vi "Main.vi"() -> ()   [LabVIEW 2015] (continued)
              n571 = case shown="False" w1144 {
                tunnel: w1143 -> [w1188 w1190]
                tunnel: [w1187 w1190] -> w1142
                frame False {
                  n572 = call "ShutterControl.vi"("error in"=w1188, "Shutter"=TRUE) -> ("error out"=w1187:errorcluster, "Status Indicator"=w1186:bool)  [unwired: 8 in]
                  n573 = local write "Shutter"(w1186) -> ()
                }
                frame True {
                }
              }
              n574 = call "ImageFrame.vi"("Tasks In"=w1184, "Vphases"=w1182, "Functions"=w1153, "error in"=w1142, "XYcoordinates"=w1183) -> ("Tasks Out"=w1180:T14, "Mixer AI Channels Data"=w1181:dbl[][], "DC AI Channel Date"=w1150:dbl[], "error out"=w1146:errorcluster)  [unwired: 6 in, 1 out]
              n575 = Unbundle By Name(w1146) -> ("status"=w1179:bool)
              n576 = Increment(x=w1157) -> (x+1=w1156:u32)
              n577 = call "Analysis.vi"("Functions"=w1153, "error in"=w1146, "Scan/Meas Parameters"=w1152, "Global Parameters"=w1151, "DC AI Channel Data"=w1150, "Mixer AI Channels Data"=w1181) -> ("AI Mix4 Data"=w1166:dbl[], "AI Mix3 Data"=w1163:dbl[], "AI Mix2 Data"=w1161:dbl[], "AI Mix1 Data"=w1159:dbl[], "AI DC Data"=w1177:dbl[], "error out"=w1145:errorcluster)
              n578 = Greater Or Equal?(x=w1156, y=w1171) -> (x >= y?=w1155:bool)
              n579 = Divide(x=w1156, y=w1171) -> (x/y=w1168:dbl)
              n580 = Compound Arithmetic op=OR(w1179, "Stop Measure", w1155) -> (w1178:bool)
              n581 = Reshape Array(w1159, w1158, w1158) -> (w1160:dbl[][])
              n582 = Reshape Array(w1161, w1158, w1158) -> (w1162:dbl[][])
              n583 = Reshape Array(w1163, w1158, w1158) -> (w1164:dbl[][])
              n584 = Reshape Array(w1166, w1158, w1158) -> (w1165:dbl[][])
              n585 = Reshape Array(w1177, w1158, w1158) -> (w1167:dbl[][])
              n586 = Multiply(x=w1168, y=100.0) -> (x*y=→"Meas Progress":dbl)
              n587 = local read "V_IF (0.5pi)"() -> (w1173:dbl[][])
              n588 = local read "V_IF (1.5pi)"() -> (w1175:dbl[][])
              n589 = local read "V_IF (pi)"() -> (w1174:dbl[][])
              n590 = local read "V_IF (0)"() -> (w1172:dbl[][])
              n591 = local read "V_DC"() -> (w1176:dbl[][])
              n592 = call "RunningAverage.vi"("New Image"=w1165, "# of Averages for the Old Image"=w1157, "Old Image"=w1175) -> ("Averaged Image"=w1138:dbl[][])  [unwired: 8 in]
              "V_IF (1.5pi)" <- w1138
              n593 = call "RunningAverage.vi"("New Image"=w1160, "# of Averages for the Old Image"=w1157, "Old Image"=w1172) -> ("Averaged Image"=w1141:dbl[][])  [unwired: 8 in]
              "V_IF (0)" <- w1141
              n594 = call "RunningAverage.vi"("New Image"=w1162, "# of Averages for the Old Image"=w1157, "Old Image"=w1173) -> ("Averaged Image"=w1140:dbl[][])  [unwired: 8 in]
              "V_IF (0.5pi)" <- w1140
              n595 = call "RunningAverage.vi"("New Image"=w1164, "# of Averages for the Old Image"=w1157, "Old Image"=w1174) -> ("Averaged Image"=w1139:dbl[][])  [unwired: 8 in]
              "V_IF (pi)" <- w1139
              n596 = call "RunningAverage.vi"("New Image"=w1167, "# of Averages for the Old Image"=w1157, "Old Image"=w1176) -> ("Averaged Image"=w1137:dbl[][])  [unwired: 8 in]
              "V_DC" <- w1137
              n597 = call "ShutterControl.vi"("error in"=w1145, "Shutter"=FALSE) -> ("error out"=w1147:errorcluster, "Status Indicator"=w1149:bool)  [unwired: 8 in]
              n598 = local write "Shutter"(w1149) -> ()
            }
            n599 = local read "[d13]"() -> (w1101:dbl)
            n600 = local read "[d24]"() -> (w1100:dbl)
            n601 = call "DAQClose.vi"("error in"=w1126, "Functions"=w1127, "Tasks In"=w1128, "DAQ Channels"=w1129) -> ("error out"=w1112:errorcluster)  [unwired: 7 in]
            n602 = local read "[M/B]"() -> (w1105:dbl)
            n603 = local read "[O_B]"() -> (w1104:dbl)
            n604 = call "GSCalculation.vi"("[d24]"=w1100, "[d13]"=w1101, "[O_B]"=w1104, "V_DC"=w1106, "[M/B]"=w1105, "V_IF (1.5pi)"=w1108, "V_IF (pi)"=w1109, "V_IF (0.5pi)"=w1110, "V_IF (0)"=w1111) -> ("S"=w1102:dbl[][], "G"=w1103:dbl[][])  [unwired: 1 in]
            "G Data" <- w1103
            "S Data" <- w1102
          }
          frame #2 {
            n605 = case shown="True" "Calculate Lifetimes and Phasors During Image Acquisition?" {
              tunnel: w1197 -> [w1200 w1229]
              tunnel: w1196 -> [_ w1221]
              tunnel: w1195 -> [_ w1208]
              tunnel: w1194 -> [_ w1207]
              tunnel: w1193 -> [_ w1206]
              tunnel: [w1200 w1201] -> w1192
              frame False {
                # "If need to be fast, e.g., 3D stack acquisition"
              }
              frame True {
                # "If do lifetime and other calcuations"
                n606 = Square(x=w1221) -> (x^2=w1239:i32)
                n607 = call "LifetimeCalculation.vi"("S"=w1206, "G"=w1207) -> ("DC&1w Lifetime"=w1230:dbl[][], "1w Lifetime"=w1231:dbl[][])  [unwired: 8 in]
                "1w Lifetime (s)" <- w1231
                "DC&1w Lifetime (s)" <- w1230
                n608 = control-ref of="1w Lifetime Hist"() -> (w1241:refnum<vi>)
                n609 = control-ref of="DC&1w Lifetime Hist"() -> (w1240:refnum<vi>)
                n610 = control-ref of="Lifetime Color Ramp"() -> (w1223:refnum<vi>)
                n611 = control-ref of="Phasor Plot"() -> (w1215:refnum<vi>)
                n612 = local read "Auto Scale?"() -> (w1203:bool)
                n613 = control-ref of="Composite Image"() -> (w1224:refnum<vi>)
                n614 = control-ref of="Image with Phasors"() -> (w1218:refnum<vi>)
                n615 = call "LifetimeHistogram.vi"("1w Lifetime"=w1231, "DC&1w Lifetime"=w1230, "1w reference"=w1241, "DC&1w reference"=w1240, "Max Lifetime (s)"="Max Lifetime (s)", "Min Lifetime (s)"="Min Lifetime (s)", "Data Size"=w1239, "error in (no error)"=w1229, "Bins"="Bins") -> ("error out"=w1225:errorcluster, "1w Lifetime Hist"=→"1w Lifetime Hist":T7, "DC&1w Lifetime Hist"=→"DC&1w Lifetime Hist":T7, "1w mean"=→"u_1w":dbl, "1w std"=→"std_1":dbl, "DC&1w mean"=→"u_01":dbl, "DC&1w std"=→"std_01":dbl)  [unwired: 4 in]
                n616 = case shown="\"1w Lifetime\", Default" "Lifetime Selection" {
                  tunnel: w1231 -> [w1245 _]
                  tunnel: w1230 -> [_ w1246]
                  tunnel: [w1245 w1246] -> w1228
                  frame "1w Lifetime", Default {
                  }
                  frame "DC&1w Lifetime" {
                  }
                }
                n617 = call "HSVCombIntensityLifetime.vi"("min_intensity"="Min Intensity", "Auto Scale?"=w1203, "max_intensity"="Max Intensity", "lifetime_max (s)"="Max Lifetime (s)", "lifetime_min (s)"="Min Lifetime (s)", "Lifetime image"=w1228, "Intensity image"=w1208) -> ("Min"=w1204:dbl, "Max"=w1205:dbl, "Lifetime Color Ramp"=→"Lifetime Color Ramp":i32[][], "HSV to RGB Picture"=→"Composite Image":picture)  [unwired: 1 in]
                n618 = call "Array2GrayPic.vi"("Pic Reference"=w1218, "Threshold (min)"=w1204, "Threshold (max)"=w1205, "Auto Scale?"=w1203, "Intensity"=w1208) -> ("Gray Picture"=→"Image with Phasors":picture)  [unwired: 6 in]
                n619 = local write "Max Intensity"(w1205) -> ()
                n620 = local write "Min Intensity"(w1204) -> ()
                n621 = property on="V_DC" class="IntGraph (strict)"(error in=w1225, "ZScale.Maximum"=w1205, "ZScale.Minimum"=w1204) -> (error out=w1222:errorcluster)  [unwired: 1 in, 1 out]
                n622 = call "CompositeProperties.vi"("Image Reference"=w1224, "Ramp Reference"=w1223, "Pixel Size"=w1221, "Max Lifetime (s)"="Max Lifetime (s)", "Min Lifetime (s)"="Min Lifetime (s)", "error in (no error)"=w1222) -> ("error out"=w1202:errorcluster)  [unwired: 13 in]
                n623 = call "DrawPhasorPlot.vi"("Intensity"=w1208, "G Data"=w1207, "S Data"=w1206, "Threshold (max)"=w1205, "Threshold (min)"=w1204, "error in"=w1202, "G_max"="G_max", "Auto Scale?"=w1203, "G_min"="G_min", "Phasor Grids"="Phasor Grids", "S_max"="S_max", "Reference"=w1215, "S_min"="S_min", "Phasor Colormap"="Phasor Colormap") -> ("Phasor Plot"=→"Phasor Plot":dbl[][], "error out"=w1201:errorcluster)  [unwired: 4 in]
              }
            }
          }
          frame #3 {
            w1254 = FALSE ("Fast Scan")
            n624 = Tick Count (ms)() -> (millisecond timer value=w1250:u32)
            n625 = local write "Measure"(w1254) -> ()
            n626 = local write "Stop Measure"(w1254) -> ()
            n627 = Subtract(x=w1250, y=w1249) -> (x-y=w1251:u32)
            n628 = To Double Precision Float(number=w1251) -> (double precision float=w1252:dbl)
            n629 = Divide(x=w1252, y=1000.0) -> (x/y=→"Actual Meas Time (s)":dbl)
          }
        }
      }
      event "Refresh": Value Change {
        n630 = event-data() -> ()  [unwired: 1 in, 1 out]
        n631 = flat-sequence {
          tunnel: [w1304] -> w1263
          tunnel: w1262 -> [w1304]
          tunnel: [w1302] -> w1260
          tunnel: w1259 -> [w1303]
          tunnel: w1263 -> [w1315]
          tunnel: [w1315] -> w1261
          tunnel: w1260 -> [w1314]
          tunnel: [w1314] -> w1258
          frame #0 {
            n632 = local read "Measurement Parameters"() -> (w1306:T4)
            n633 = Unbundle By Name(w1306) -> ("Pixel Size"=w1305:dbl)
            n634 = local read "G Data"() -> (w1308:dbl[][])
            n635 = local read "V_DC"() -> (w1310:dbl[][])
            n636 = local read "S Data"() -> (w1309:dbl[][])
            n637 = To Long Integer(number=w1305) -> (32bit integer=w1307:i32)
            n638 = Square(x=w1307) -> (x^2=w1301:i32)
            n639 = local read "Phasor Colormap"() -> (w1266:T8)
            n640 = local read "Max Lifetime (s)"() -> (w1295:dbl)
            n641 = local read "Min Lifetime (s)"() -> (w1294:dbl)
            n642 = control-ref of="Phasor Plot"() -> (w1265:refnum<vi>)
            n643 = control-ref of="Lifetime Color Ramp"() -> (w1275:refnum<vi>)
            n644 = call "LifetimeCalculation.vi"("S"=w1309, "G"=w1308) -> ("DC&1w Lifetime"=w1290:dbl[][], "1w Lifetime"=w1291:dbl[][])  [unwired: 8 in]
            n645 = local read "Bins"() -> (w1289:i32)
            n646 = control-ref of="1w Lifetime Hist"() -> (w1282:refnum<vi>)
            n647 = control-ref of="DC&1w Lifetime Hist"() -> (w1281:refnum<vi>)
            n648 = local read "Phasor Grids"() -> (w1267:i32)
            n649 = local read "Max Intensity"() -> (w1293:dbl)
            n650 = local read "Min Intensity"() -> (w1292:dbl)
            n651 = local read "Auto Scale?"() -> (w1297:bool)
            n652 = local read "G_max"() -> (w1271:dbl)
            n653 = local read "G_min"() -> (w1270:dbl)
            n654 = local read "S_max"() -> (w1269:dbl)
            n655 = local read "S_min"() -> (w1268:dbl)
            n656 = control-ref of="Image with Phasors"() -> (w1274:refnum<vi>)
            n657 = control-ref of="Composite Image"() -> (w1276:refnum<vi>)
            n658 = call "LifetimeHistogram.vi"("1w Lifetime"=w1291, "DC&1w Lifetime"=w1290, "1w reference"=w1282, "DC&1w reference"=w1281, "Max Lifetime (s)"=w1295, "Min Lifetime (s)"=w1294, "Data Size"=w1301, "error in (no error)"=w1303, "Bins"=w1289) -> ("error out"=w1299:errorcluster, "1w Lifetime Hist"=w1288:T7, "DC&1w Lifetime Hist"=w1287:T7, "1w mean"=w1286:dbl, "1w std"=w1285:dbl, "DC&1w mean"=w1284:dbl, "DC&1w std"=w1283:dbl)  [unwired: 4 in]
            n659 = local write "1w Lifetime (s)"(w1291) -> ()
            n660 = local write "DC&1w Lifetime (s)"(w1290) -> ()
            n661 = local write "1w Lifetime Hist"(w1288) -> ()
            n662 = local write "DC&1w Lifetime Hist"(w1287) -> ()
            n663 = local write "u_1w"(w1286) -> ()
            n664 = local write "std_1"(w1285) -> ()
            n665 = local write "u_01"(w1284) -> ()
            n666 = local write "std_01"(w1283) -> ()
            n667 = local read "Lifetime Selection"() -> (w1264:enum32{"1w Lifetime", "DC&1w Lifetime"})
            n668 = case shown="\"1w Lifetime\", Default" w1264 {
              tunnel: w1291 -> [w1311 _]
              tunnel: w1290 -> [_ w1312]
              tunnel: [w1311 w1312] -> w1300
              frame "1w Lifetime", Default {
              }
              frame "DC&1w Lifetime" {
              }
            }
            n669 = call "HSVCombIntensityLifetime.vi"("min_intensity"=w1292, "Auto Scale?"=w1297, "max_intensity"=w1293, "lifetime_max (s)"=w1295, "lifetime_min (s)"=w1294, "Lifetime image"=w1300, "Intensity image"=w1310) -> ("Min"=w1277:dbl, "Max"=w1278:dbl, "Lifetime Color Ramp"=w1279:i32[][], "HSV to RGB Picture"=w1280:picture)  [unwired: 1 in]
            n670 = call "Array2GrayPic.vi"("Pic Reference"=w1274, "Threshold (min)"=w1277, "Threshold (max)"=w1278, "Auto Scale?"=w1297, "Intensity"=w1310) -> ("Gray Picture"=w1273:picture)  [unwired: 6 in]
            n671 = local write "Image with Phasors"(w1273) -> ()
            n672 = property on="V_DC" class="IntGraph (strict)"(error in=w1299, "ZScale.Maximum"=w1278, "ZScale.Minimum"=w1277) -> (error out=w1298:errorcluster)  [unwired: 1 in, 1 out]
            n673 = call "CompositeProperties.vi"("Image Reference"=w1276, "Ramp Reference"=w1275, "Pixel Size"=w1307, "Max Lifetime (s)"=w1295, "Min Lifetime (s)"=w1294, "error in (no error)"=w1298) -> ("error out"=w1296:errorcluster)  [unwired: 13 in]
            n674 = call "DrawPhasorPlot.vi"("Intensity"=w1310, "G Data"=w1308, "S Data"=w1309, "Threshold (max)"=w1278, "Threshold (min)"=w1277, "error in"=w1296, "G_max"=w1271, "Auto Scale?"=w1297, "G_min"=w1270, "Phasor Grids"=w1267, "S_max"=w1269, "Reference"=w1265, "S_min"=w1268, "Phasor Colormap"=w1266) -> ("Phasor Plot"=w1272:dbl[][], "error out"=w1302:errorcluster)  [unwired: 4 in]
            n675 = local write "Phasor Plot"(w1272) -> ()
            n676 = local write "Composite Image"(w1280) -> ()
            n677 = local write "Lifetime Color Ramp"(w1279) -> ()
            n678 = local write "Max Intensity"(w1278) -> ()
            n679 = local write "Min Intensity"(w1277) -> ()
          }
          frame #1 {
            n680 = local write "Refresh"(FALSE ("Fast Scan")) -> ()
          }
        }
      }
      event "Z-Stack Measure": Value Change {
        n681 = event-data() -> ()  [unwired: 1 in, 1 out]
        n682 = local read "Current Slice"() -> (w1324:i32)
        n683 = Divide(x=w1324, y="Z Slice Number") -> (x/y=w1332:dbl)
        n684 = Greater Or Equal?(x=w1324, y="Z Slice Number") -> (x >= y?=w1325:bool)
        n685 = Multiply(x=w1332, y=100.0) -> (x*y=→"Stack Progress":dbl)
        n686 = Equal To 0?(x=w1324) -> (x = 0?=w1323:bool)
        n687 = case shown="False" w1323 {
          tunnel: w1334 -> [w1380 w1407]
          tunnel: w1335 -> [w1379 w1408]
          tunnel: [w1378 w1406] -> w1328
          tunnel: [w1377 w1405] -> w1326
          tunnel: w1325 -> [w1373 _]
          tunnel: [FALSE ("Stop Stack Measure") w1400] -> w1316
          frame False {
            # "Continue measurement , move stage"
            n688 = local read "3D Intensity"() -> (w1374:dbl[][][])
            n689 = local read "G Data"() -> (w1372:dbl[][])
            n690 = local read "S Data"() -> (w1371:dbl[][])
            n691 = local read "V_DC"() -> (w1376:dbl[][])
            n692 = local read "3D G"() -> (w1368:dbl[][][])
            n693 = local read "3D S"() -> (w1367:dbl[][][])
            n694 = case shown="False" w1373 {
              tunnel: w1380 -> [w1396 w1397]
              tunnel: w1379 -> [w1395 w1398]
              tunnel: [w1383 w1398] -> w1378
              tunnel: [w1381 w1397] -> w1377
              frame False {
                # "Moves up by 1 step defined by \nthe 'C' command"
                n695 = Number To Decimal String(number="Z Slice Size (.1um)") -> (decimal integer string=w1389:string)  [unwired: 1 in]
                n696 = Concatenate Strings("C" ("string"), "," ("string"), w1389, "\r", "U" ("string")) -> (w1386:string)
                n697 = VISA Write(VISA resource name=w1395, write buffer=w1386, error in (no error)=w1396) -> (VISA resource name out=w1393:refnum<visa-resource-name>, error out=w1392:errorcluster)  [unwired: 1 out]
                n698 = VISA Read(VISA resource name=w1393, byte count=u32 256, error in (no error)=w1392) -> (VISA resource name out=w1384:refnum<visa-resource-name>, error out=w1382:errorcluster)  [unwired: 2 out]
                n699 = VISA Clear(VISA resource name=w1384, error in (no error)=w1382) -> (VISA resource name out=w1383:refnum<visa-resource-name>, error out=w1381:errorcluster)
              }
              frame True {
              }
            }
            n700 = Build Array (concatenate)(w1374, w1376) -> (→"3D Intensity":dbl[][][])
            n701 = Build Array (concatenate)(w1368, w1372) -> (→"3D G":dbl[][][])
            n702 = Build Array (concatenate)(w1367, w1371) -> (→"3D S":dbl[][][])
          }
          frame True {
            # "Beginning the measurment, record current Z position"
            n703 = local read "3D Time-Lapse Measure"() -> (w1399:bool)
            n704 = case shown="False" w1399 {
              tunnel: [w1413 TRUE ("T button?")] -> w1401
              frame False {
                n705 = Two Button Dialog(message="Discard Previous Stack?") -> (T button?=w1413:bool)  [unwired: 2 in]
              }
              frame True {
              }
            }
            n706 = local write "Calculate Lifetimes and Phasors During Image Acquisition?"(FALSE ("Calculate Lifetimes and Phasors During Image Acquisition?")) -> ()
            n707 = VISA Write(VISA resource name=w1408, write buffer="PZ" ("string"), error in (no error)=w1407) -> (VISA resource name out=w1410:refnum<visa-resource-name>, error out=w1411:errorcluster)  [unwired: 1 out]
            n708 = VISA Read(VISA resource name=w1410, byte count=u32 256, error in (no error)=w1411) -> (VISA resource name out=w1406:refnum<visa-resource-name>, read buffer=w1404:string, error out=w1405:errorcluster)  [unwired: 1 out]
            n709 = case shown="True" w1401 {
              tunnel: [TRUE ("Stop Stack Measure") FALSE ("Stop Stack Measure")] -> w1400
              frame False {
              }
              frame True {
                w1418 = dbl[][][] [] ("3D Intensity (BT)")
                n710 = local write "3D Intensity"(w1418) -> ()
                n711 = local write "3D G"(w1418) -> ()
                n712 = local write "3D S"(w1418) -> ()
              }
            }
            n713 = Decimal String To Number(string=w1404) -> (number=→"Initial Z Pos (.1um)":i32)  [unwired: 2 in, 1 out]
          }
        }
        n714 = Compound Arithmetic op=OR(w1325, "Stop Stack Measure", w1316) -> (w1329:bool)
        n715 = case shown="True" w1329 {
          tunnel: w1328 -> [w1342 w1346]
          tunnel: w1326 -> [w1337 w1345]
          tunnel: [w1342 w1351] -> w1322
          tunnel: [w1339 w1347] -> w1320
          tunnel: w1324 -> [w1341 _]
          frame False {
            n716 = Increment(x=w1341) -> (x+1=→"Current Slice":i32)
            n717 = property on="Measure" class="Bool (strict)"(error in=w1337, "Val(Sgnl)"=TRUE ("Value (Signaling)")) -> (error out=w1336:errorcluster)  [unwired: 1 in, 1 out]
            n718 = property on="Z-Stack Measure" class="Bool (strict)"(error in=w1336, "Val(Sgnl)"=TRUE ("Value (Signaling)")) -> (error out=w1339:errorcluster)  [unwired: 1 in, 1 out]
          }
          frame True {
            w1350 = FALSE ("Fast Scan")
            n719 = local read "Initial Z Pos (.1um)"() -> (w1360:i32)
            n720 = local read "3D Time-Lapse Measure"() -> (w1349:bool)
            n721 = local write "Calculate Lifetimes and Phasors During Image Acquisition?"(TRUE ("Calculate Lifetimes and Phasors During Image Acquisition?")) -> ()
            n722 = local write "Stop Stack Measure"(w1350) -> ()
            n723 = local write "Z-Stack Measure"(w1350) -> ()
            n724 = local write "Current Slice"(0 ("Current Slice")) -> ()
            n725 = Number To Decimal String(number=w1360) -> (decimal integer string=w1357:string)  [unwired: 1 in]
            n726 = Concatenate Strings("GZ" ("string"), "," ("string"), w1357) -> (w1359:string)
            n727 = VISA Write(VISA resource name=w1346, write buffer=w1359, error in (no error)=w1345) -> (VISA resource name out=w1354:refnum<visa-resource-name>, error out=w1355:errorcluster)  [unwired: 1 out]
            n728 = VISA Read(VISA resource name=w1354, byte count=u32 256, error in (no error)=w1355) -> (VISA resource name out=w1351:refnum<visa-resource-name>, error out=w1348:errorcluster)  [unwired: 2 out]
            n729 = case shown="True" w1349 {
              tunnel: w1348 -> [w1361 w1363]
              tunnel: [w1361 w1362] -> w1347
              frame False {
              }
              frame True {
                w1364 = TRUE ("Value (Signaling)")
                n730 = property on="Save 3D Stacks" class="Bool (strict)"(error in=w1363, "Val(Sgnl)"=w1364) -> (error out=w1365:errorcluster)  [unwired: 1 in, 1 out]
                n731 = property on="3D Time-Lapse Measure" class="Bool (strict)"(error in=w1365, "Val(Sgnl)"=w1364) -> (error out=w1362:errorcluster)  [unwired: 1 in, 1 out]
              }
            }
          }
        }
        n732 = VISA Clear(VISA resource name=w1322, error in (no error)=w1320) -> (VISA resource name out=w1321:refnum<visa-resource-name>, error out=w1319:errorcluster)
      }
      event "3D Stack to Show", "Slice Slider": Value Change {
        n733 = event-data() -> ()  [unwired: 1 in, 1 out]
        n734 = local read "3D Intensity"() -> (w1441:dbl[][][])
        n735 = local read "Max Lifetime (s)"() -> (w1443:dbl)
        n736 = local read "Min Lifetime (s)"() -> (w1442:dbl)
        n737 = case shown="False" "Auto Scale?" {
          tunnel: w1441 -> [_ w1461]
          tunnel: [w1458 w1460] -> w1440
          tunnel: [w1457 w1459] -> w1439
          frame False {
            n738 = local read "Max Intensity"() -> (w1458:dbl)
            n739 = local read "Min Intensity"() -> (w1457:dbl)
          }
          frame True {
            n740 = Array Max & Min(array=w1461) -> (max value=w1460:dbl, min value=w1459:dbl)  [unwired: 2 out]
          }
        }
        n741 = local read "3D G"() -> (w1425:dbl[][][])
        n742 = local read "3D S"() -> (w1424:dbl[][][])
        n743 = control-ref of="Slice of 3D Stack"() -> (w1426:refnum<vi>)
        n744 = Multiply(x=80000000.0, y=6.283185307179586) -> (x*y=w1421:dbl)
        n745 = case shown="\"Intensity 3D\", Default" "3D Stack to Show" {
          tunnel: "Slice Slider" -> [w1471 w1484 w1500 w1517 w1538 w1558 w1577]
          tunnel: [w1469 w1483 w1499 w1518 w1537 w1561 w1580] -> w1444
          tunnel: w1443 -> [_ w1479 w1496 w1510 w1528 _ _]
          tunnel: w1442 -> [_ w1478 w1495 w1509 w1521 _ _]
          tunnel: w1441 -> [w1468 _ _ w1516 w1536 w1562 w1581]
          tunnel: w1440 -> [w1464 _ _ w1513 w1531 w1547 w1572]
          tunnel: w1439 -> [w1463 _ _ w1512 w1530 w1546 w1571]
          tunnel: [w1462 w1477 w1494 w1507 w1533 w1542 w1574] -> w1428
          tunnel: w1426 -> [w1466 w1481 w1493 w1515 w1534 w1543 w1576]
          tunnel: w1425 -> [_ w1475 w1490 w1505 w1523 w1560 w1579]
          tunnel: w1424 -> [_ w1474 _ w1504 _ w1559 w1578]
          tunnel: w1421 -> [_ w1473 w1487 w1503 w1522 _ _]
          frame "Intensity 3D", Default {
            n746 = Array Size(array=w1468) -> (size(s)=w1470:i32[])
            n747 = Index Array(array=w1468, index (dim 0)=w1471) -> (element=w1467:dbl[][])  [unwired: 2 in]
            n748 = Index Array(array=w1470) -> (element=w1469:i32)  [unwired: 1 in]
            n749 = call "Array2GrayPic.vi"("Pic Reference"=w1466, "Threshold (min)"=w1463, "Threshold (max)"=w1464, "Auto Scale?"=FALSE, "Intensity"=w1467) -> ("Gray Picture"=w1462:picture)  [unwired: 6 in]
          }
          frame "1w Lifetime 3D" {
            n750 = Divide(x=w1474, y=w1475) -> (x/y=w1476:dbl[][][])
            n751 = Divide(x=w1476, y=w1473) -> (x/y=w1472:dbl[][][])
            n752 = Array Size(array=w1472) -> (size(s)=w1485:i32[])
            n753 = Index Array(array=w1472, index (dim 0)=w1484) -> (element=w1480:dbl[][])  [unwired: 2 in]
            n754 = Index Array(array=w1485) -> (element=w1483:i32)  [unwired: 1 in]
            n755 = call "Array2GrayPic.vi"("Pic Reference"=w1481, "Threshold (min)"=w1478, "Threshold (max)"=w1479, "Auto Scale?"=FALSE, "Intensity"=w1480) -> ("Gray Picture"=w1477:picture)  [unwired: 6 in]
          }
          frame "DC&1w Lifetime 3D" {
            n756 = Divide(x=1.0, y=w1490) -> (x/y=w1489:dbl[][][])
            n757 = Decrement(x=w1489) -> (x-1=w1492:dbl[][][])
            n758 = Square Root(x=w1492) -> (sqrt(x)=w1488:dbl[][][])
            n759 = Divide(x=w1488, y=w1487) -> (x/y=w1486:dbl[][][])
            n760 = Array Size(array=w1486) -> (size(s)=w1501:i32[])
            n761 = Index Array(array=w1486, index (dim 0)=w1500) -> (element=w1497:dbl[][])  [unwired: 2 in]
            n762 = Index Array(array=w1501) -> (element=w1499:i32)  [unwired: 1 in]
            n763 = call "Array2GrayPic.vi"("Pic Reference"=w1493, "Threshold (min)"=w1495, "Threshold (max)"=w1496, "Auto Scale?"=FALSE, "Intensity"=w1497) -> ("Gray Picture"=w1494:picture)  [unwired: 6 in]
          }
          frame "1w Composite 3D" {
            n764 = Divide(x=w1504, y=w1505) -> (x/y=w1506:dbl[][][])
            n765 = Divide(x=w1506, y=w1503) -> (x/y=w1502:dbl[][][])
            n766 = Index Array(array=w1502, index (dim 0)=w1517) -> (element=w1511:dbl[][])  [unwired: 2 in]
            n767 = Index Array(array=w1516, index (dim 0)=w1517) -> (element=w1514:dbl[][])  [unwired: 2 in]
            n768 = Array Size(array=w1516) -> (size(s)=w1519:i32[])
            n769 = Index Array(array=w1519) -> (element=w1518:i32)  [unwired: 1 in]
            n770 = call "Array2HSVColorPic.vi"("Intensity"=w1514, "Threshold (max)"=w1513, "Threshold (min)"=w1512, "Lifetime"=w1511, "lifetime_max (s)"=w1510, "lifetime_min (s)"=w1509, "Pic Reference"=w1515, "Auto Scale?"=FALSE) -> ("Gray Picture"=w1507:picture)  [unwired: 11 in]
          }
          frame "DC&1w Composite 3D" {
            n771 = Divide(x=1.0, y=w1523) -> (x/y=w1525:dbl[][][])
            n772 = Decrement(x=w1525) -> (x-1=w1527:dbl[][][])
            n773 = Square Root(x=w1527) -> (sqrt(x)=w1524:dbl[][][])
            n774 = Divide(x=w1524, y=w1522) -> (x/y=w1520:dbl[][][])
            n775 = Index Array(array=w1520, index (dim 0)=w1538) -> (element=w1529:dbl[][])  [unwired: 2 in]
            n776 = Index Array(array=w1536, index (dim 0)=w1538) -> (element=w1532:dbl[][])  [unwired: 2 in]
            n777 = Array Size(array=w1536) -> (size(s)=w1539:i32[])
            n778 = Index Array(array=w1539) -> (element=w1537:i32)  [unwired: 1 in]
            n779 = call "Array2HSVColorPic.vi"("Intensity"=w1532, "Threshold (max)"=w1531, "Threshold (min)"=w1530, "Lifetime"=w1529, "lifetime_max (s)"=w1528, "lifetime_min (s)"=w1521, "Pic Reference"=w1534, "Auto Scale?"=FALSE) -> ("Gray Picture"=w1533:picture)  [unwired: 11 in]
          }
          frame "Phasor 3D" {
            # "Transpose"
            n780 = Array Size(array=w1562) -> (size(s)=w1563:i32[])
            n781 = Index Array(array=w1559, index (dim 0)=w1558) -> (element=w1548:dbl[][])  [unwired: 2 in]
            n782 = Index Array(array=w1560, index (dim 0)=w1558) -> (element=w1549:dbl[][])  [unwired: 2 in]
            n783 = Index Array(array=w1562, index (dim 0)=w1558) -> (element=w1550:dbl[][])  [unwired: 2 in]
            n784 = Index Array(array=w1563) -> (element=w1561:i32)  [unwired: 1 in]
            n785 = local read "Phasor Colormap"() -> (w1551:T8)
            n786 = local read "G_max"() -> (w1557:dbl)
            n787 = local read "G_min"() -> (w1556:dbl)
            n788 = local read "S_max"() -> (w1555:dbl)
            n789 = local read "S_min"() -> (w1554:dbl)
            n790 = control-ref of="Phasor Plot"() -> (w1552:refnum<vi>)
            n791 = local read "Phasor Grids"() -> (w1553:i32)
            n792 = call "DrawPhasorPlot.vi"("Intensity"=w1550, "G Data"=w1549, "S Data"=w1548, "Threshold (max)"=w1547, "Threshold (min)"=w1546, "G_max"=w1557, "Auto Scale?"=FALSE, "G_min"=w1556, "Phasor Grids"=w1553, "S_max"=w1555, "Reference"=w1552, "S_min"=w1554, "Phasor Colormap"=w1551) -> ("Phasor Plot"=w1540:dbl[][])  [unwired: 5 in, 1 out]
            n793 = Transpose 2D Array(2D array=w1540) -> (transposed array=w1541:dbl[][])
            n794 = call "Array2GrayPic.vi"("Pic Reference"=w1543, "Auto Scale?"=TRUE, "Intensity"=w1541) -> ("Gray Picture"=w1542:picture)  [unwired: 8 in]
          }
          frame "Overlap 3D" {
            n795 = Array Size(array=w1581) -> (size(s)=w1582:i32[])
            n796 = Index Array(array=w1581, index (dim 0)=w1577) -> (element=w1575:dbl[][])  [unwired: 2 in]
            n797 = Index Array(array=w1578, index (dim 0)=w1577) -> (element=w1569:dbl[][])  [unwired: 2 in]
            n798 = Index Array(array=w1579, index (dim 0)=w1577) -> (element=w1570:dbl[][])  [unwired: 2 in]
            n799 = Index Array(array=w1582) -> (element=w1580:i32)  [unwired: 1 in]
            n800 = local read "ROI Cluster"() -> (w1568:T9)
            n801 = Unbundle(w1568) -> (w1567:bool[], w1566:dbl[], w1565:cluster{dbl, dbl}[], w1564:u32[])
            n802 = call "PhasorROI2IMG.vi"("Intensity"=w1575, "Auto Scale?"=FALSE, "Threshold (max)"=w1572, "Threshold (min)"=w1571, "G Data"=w1570, "S Data"=w1569, "Pic Reference"=w1576, "ROI? array"=w1567, "Radius array"=w1566, "Center array"=w1565, "Color array"=w1564) -> ("new picture"=w1574:picture)  [unwired: 8 in]
          }
        }
        "Slice of 3D Stack" <- w1428
        "Number of Slices" <- w1444
        n803 = local read "Measurement Parameters"() -> (w1438:T4)
        n804 = property on="Slice of 3D Stack" class="Pict"(error in=w1432) -> (error out=w1431:errorcluster, "Draw Area Size"=w1436:T16)  [unwired: 1 in, 1 out]
        n805 = Unbundle By Name(w1436) -> ("Width"=w1433:u32)
        n806 = Unbundle By Name(w1438) -> ("Pixel Size"=w1429:dbl)
        n807 = To Single Precision Float(number=w1433) -> (single precision float=w1435:sgl)
        n808 = To Single Precision Float(number=w1429) -> (single precision float=w1434:sgl)
        n809 = Divide(x=w1435, y=w1434) -> (x/y=w1437:sgl)
        n810 = property on="Slice of 3D Stack" class="Pict"(error in=w1431, "ZoomFactor"=w1437) -> (error out=w1430:errorcluster)  [unwired: 1 in, 1 out]
        n811 = Increment(x="Slice Slider") -> (x+1=w1450:i32)
        n812 = Number To Decimal String(number=w1450) -> (decimal integer string=w1448:string)  [unwired: 1 in]
        n813 = Number To Decimal String(number=w1444) -> (decimal integer string=w1453:string)  [unwired: 1 in]
        n814 = property on="Slice Slider" class="Scroll (strict)"(error in=w1430, "DocMax"=w1444) -> (error out=w1447:errorcluster)  [unwired: 1 in, 1 out]
        n815 = Concatenate Strings("Slice #: " ("string"), w1448, "/" ("string"), w1453) -> (→"Slice Display":string)
        n816 = property on="Slice Slider" class="Scroll (strict)"(error in=w1447, "DocMin"=0.0 ("Doc Min")) -> (error out=w1446:errorcluster)  [unwired: 1 in, 1 out]
      }
      event "Save 3D Stacks": Value Change {
        # "Always save raw data for 3D"
        n817 = event-data() -> ()  [unwired: 1 in, 1 out]
        n818 = local read "3D Intensity"() -> (w1611:dbl[][][])
        n819 = local read "Current 3D Time-Lapse Meas"() -> (w1613:i32)
        n820 = local read "Crop Pixels"() -> (w1598:u16)
        n821 = local read "3D G"() -> (w1603:dbl[][][])
        n822 = local read "3D S"() -> (w1601:dbl[][][])
        n823 = case shown="True" TRUE {
          tunnel: [w1617 w1619] -> w1610
          tunnel: [w1616 w1618] -> w1609
          tunnel: w1611 -> [_ w1620]
          frame False {
            n824 = local read "Max Intensity"() -> (w1617:dbl)
            n825 = local read "Min Intensity"() -> (w1616:dbl)
          }
          frame True {
            n826 = Array Max & Min(array=w1620) -> (max value=w1619:dbl, min value=w1618:dbl)  [unwired: 2 out]
          }
        }
        n827 = case shown="True" "Current Directory (3D)?" {
          tunnel: ["Save Directory (3D)" w1622] -> w1599
          frame False {
          }
          frame True {
            n828 = Current VI's Path() -> (path=w1623:path)
            n829 = Strip Path(path=w1623) -> (stripped path=w1622:path)  [unwired: 1 out]
          }
        }
        n830 = Number To Decimal String(number=w1613) -> (decimal integer string=w1596:string)  [unwired: 1 in]
        n831 = call "Save3DStack.vi"("Experiment Name"="Experiment Name (3D)", "Identify Name"="I" ("string"), "3D Data"=w1611, "matrix_max"=w1610, "matrix_min"=w1609, "error in"=w1608, "File Name"="File Name (3D)", "Index Name"=w1596, "path"=w1599, "Specify Range?"=TRUE ("Bound Pixel Value?"), "Enable?"=TRUE, "Crop Pixels"=w1598, "Time Stamp?"=FALSE ("Enable?")) -> ("error out"=w1604:errorcluster)  [unwired: 5 in, 1 out]
        n832 = call "Save3DStack.vi"("Experiment Name"="Experiment Name (3D)", "Identify Name"="G" ("string"), "3D Data"=w1603, "error in"=w1604, "File Name"="File Name (3D)", "Index Name"=w1596, "path"=w1599, "Specify Range?"=FALSE ("Bound Pixel Value?"), "Enable?"=TRUE, "Crop Pixels"=w1598, "Time Stamp?"=FALSE ("Enable?")) -> ("error out"=w1591:errorcluster)  [unwired: 7 in, 1 out]
        n833 = call "Save3DStack.vi"("Experiment Name"="Experiment Name (3D)", "Identify Name"="S" ("string"), "3D Data"=w1601, "error in"=w1591, "File Name"="File Name (3D)", "Index Name"=w1596, "path"=w1599, "Specify Range?"=FALSE ("Bound Pixel Value?"), "Enable?"=TRUE, "Crop Pixels"=w1598, "Time Stamp?"=FALSE ("Enable?")) -> ("error out"=w1602:errorcluster)  [unwired: 7 in, 1 out]
        n834 = flat-sequence {
          tunnel: w1602 -> [w1625]
          tunnel: [w1625] -> w1586
          frame #0 {
            n835 = local write "Save 3D Stacks"(FALSE ("Save 3D Stacks")) -> ()
          }
        }
      }
      event "2D Time-Lapse Measure": Value Change {
        n836 = event-data() -> ()  [unwired: 1 in, 1 out]
        n837 = local read "Current 2D Time-Lapse Meas"() -> (w1631:i32)
        n838 = Divide(x=w1631, y="Total 2D Time-Lapse Meas") -> (x/y=w1636:dbl)
        n839 = Greater Or Equal?(x=w1631, y="Total 2D Time-Lapse Meas") -> (x >= y?=w1637:bool)
        n840 = Multiply(x=w1636, y=100.0) -> (x*y=→"2D Time-Lapse Progress":dbl)
        n841 = Compound Arithmetic op=OR(w1637, "Stop 2D Time-Lapse") -> (w1633:bool)
        n842 = case shown="False" w1633 {
          tunnel: w1631 -> [w1642 _]
          tunnel: w1629 -> [w1643 w1662]
          tunnel: [w1644 w1662] -> w1628
          frame False {
            w1645 = TRUE ("Value (Signaling)")
            n843 = Equal To 0?(x=w1642) -> (x = 0?=w1641:bool)
            n844 = case shown="False" w1641 {
              tunnel: [w1652 w1661] -> w1640
              tunnel: w1643 -> [w1652 w1661]
              frame False {
                n845 = while {
                  stop <- w1654 stop-if-true
                  n846 = local read "Time Stamp (s)"() -> (w1658:dbl)
                  n847 = Get Date/Time In Seconds() -> (seconds since 1Jan1904=w1660:timestamp)
                  n848 = local read "Stop 2D Time-Lapse"() -> (w1653:bool)
                  n849 = To Double Precision Float(number=w1660) -> (double precision float=w1659:dbl)
                  n850 = Subtract(x=w1659, y=w1658) -> (x-y=w1657:dbl)
                  "Time Elapse (s)" <- w1657
                  n851 = Greater Or Equal?(x=w1657, y="2D Time-Lapse Interval (s)") -> (x >= y?=w1655:bool)
                  n852 = Compound Arithmetic op=OR(w1655, w1653) -> (w1654:bool)
                }
              }
              frame True {
              }
            }
            n853 = Increment(x=w1642) -> (x+1=→"Current 2D Time-Lapse Meas":i32)
            n854 = flat-sequence {
              tunnel: [w1651] -> w1639
              tunnel: w1640 -> [w1651]
              frame #0 {
                n855 = Get Date/Time In Seconds() -> (seconds since 1Jan1904=w1649:timestamp)
                n856 = To Double Precision Float(number=w1649) -> (double precision float=→"Time Stamp (s)":dbl)
              }
            }
            n857 = property on="Measure" class="Bool (strict)"(error in=w1639, "Val(Sgnl)"=w1645) -> (error out=w1647:errorcluster)  [unwired: 1 in, 1 out]
            n858 = property on="Save 2D Images" class="Bool (strict)"(error in=w1647, "Val(Sgnl)"=w1645) -> (error out=w1646:errorcluster)  [unwired: 1 in, 1 out]
            n859 = property on="2D Time-Lapse Measure" class="Bool (strict)"(error in=w1646, "Val(Sgnl)"=w1645) -> (error out=w1644:errorcluster)  [unwired: 1 in, 1 out]
          }
          frame True {
            w1663 = FALSE ("2D Time-Lapse Measure")
            n860 = local write "Current 2D Time-Lapse Meas"(0 ("Current Slice")) -> ()
            n861 = local write "2D Time-Lapse Measure"(w1663) -> ()
            n862 = local write "Stop 2D Time-Lapse"(w1663) -> ()
          }
        }
      }
      event "3D Time-Lapse Measure": Value Change {
        n863 = event-data() -> ()  [unwired: 1 in, 1 out]
        n864 = local read "Current 3D Time-Lapse Meas"() -> (w1675:i32)
        n865 = Divide(x=w1675, y="Total 3D Time-Lapse Meas") -> (x/y=w1669:dbl)
        n866 = Greater Or Equal?(x=w1675, y="Total 3D Time-Lapse Meas") -> (x >= y?=w1673:bool)
        n867 = Multiply(x=w1669, y=100.0) -> (x*y=→"3D Time-Lapse Progress":dbl)
        n868 = Compound Arithmetic op=OR(w1673, "Stop 3D Time-Lapse") -> (w1676:bool)
        n869 = case shown="False" w1676 {
          tunnel: w1675 -> [w1684 _]
          tunnel: w1668 -> [w1681 w1699]
          tunnel: [w1678 w1699] -> w1667
          frame False {
            n870 = Equal To 0?(x=w1684) -> (x = 0?=w1683:bool)
            n871 = case shown="False" w1683 {
              tunnel: w1681 -> [w1689 w1698]
              tunnel: [w1689 w1698] -> w1680
              frame False {
                n872 = while {
                  stop <- w1690 stop-if-true
                  n873 = local read "Time Stamp (s)"() -> (w1695:dbl)
                  n874 = Get Date/Time In Seconds() -> (seconds since 1Jan1904=w1697:timestamp)
                  n875 = local read "Stop 3D Time-Lapse"() -> (w1691:bool)
                  n876 = To Double Precision Float(number=w1697) -> (double precision float=w1696:dbl)
                  n877 = Subtract(x=w1696, y=w1695) -> (x-y=w1693:dbl)
                  n878 = Greater Or Equal?(x=w1693, y="3D Time-Lapse Interval (s)") -> (x >= y?=w1694:bool)
                  n879 = local write "Time Elapse (s)"(w1693) -> ()
                  n880 = Compound Arithmetic op=OR(w1694, w1691) -> (w1690:bool)
                }
              }
              frame True {
              }
            }
            n881 = Increment(x=w1684) -> (x+1=→"Current 3D Time-Lapse Meas":i32)
            n882 = flat-sequence {
              tunnel: [w1686] -> w1679
              tunnel: w1680 -> [w1686]
              frame #0 {
                n883 = Get Date/Time In Seconds() -> (seconds since 1Jan1904=w1688:timestamp)
                n884 = To Double Precision Float(number=w1688) -> (double precision float=w1687:dbl)
                n885 = local write "Time Stamp (s)"(w1687) -> ()
              }
            }
            n886 = property on="Z-Stack Measure" class="Bool (strict)"(error in=w1679, "Val(Sgnl)"=TRUE ("Value (Signaling)")) -> (error out=w1678:errorcluster)  [unwired: 1 in, 1 out]
          }
          frame True {
            w1700 = FALSE ("2D Time-Lapse Measure")
            n887 = local write "Current 3D Time-Lapse Meas"(0 ("Current Slice")) -> ()
            n888 = local write "3D Time-Lapse Measure"(w1700) -> ()
            n889 = local write "Stop 3D Time-Lapse"(w1700) -> ()
          }
        }
      }
      event "Lifetime Selection", "Min Lifetime (s)", "Max Lifetime (s)", "Bins", "Max Intensity", "Min Intensity", "Auto Scale?": Value Change {
        w1717 = 100.0 ("y")
        n890 = event-data() -> ()  [unwired: 1 in, 1 out]
        n891 = local read "Lifetime Selection"() -> (w1743:enum32{"1w Lifetime", "DC&1w Lifetime"})
        n892 = case shown="\"DC&1w Lifetime\"" w1743 {
          tunnel: [w1745 w1746] -> w1738
          frame "1w Lifetime", Default {
            n893 = local read "1w Lifetime (s)"() -> (w1745:dbl[][])
          }
          frame "DC&1w Lifetime" {
            n894 = local read "DC&1w Lifetime (s)"() -> (w1746:dbl[][])
          }
        }
        n895 = local read "Auto Scale?"() -> (w1735:bool)
        n896 = local read "Max Lifetime (s)"() -> (w1712:dbl)
        n897 = local read "Max Intensity"() -> (w1737:dbl)
        n898 = local read "Min Lifetime (s)"() -> (w1711:dbl)
        n899 = local read "Min Intensity"() -> (w1736:dbl)
        n900 = local read "V_DC"() -> (w1727:dbl[][])
        n901 = call "HSVCombIntensityLifetime.vi"("min_intensity"=w1736, "Auto Scale?"=w1735, "max_intensity"=w1737, "lifetime_max (s)"=w1712, "lifetime_min (s)"=w1711, "Lifetime image"=w1738, "Intensity image"=w1727) -> ("Min"=w1704:dbl, "Max"=w1705:dbl, "Lifetime Color Ramp"=w1742:i32[][], "HSV to RGB Picture"=w1741:picture)  [unwired: 1 in]
        n902 = Array Max & Min(array=w1727) -> (max value=w1726:dbl, min value=w1724:dbl)  [unwired: 2 out]
        n903 = local write "Lifetime Color Ramp"(w1742) -> ()
        n904 = local write "Composite Image"(w1741) -> ()
        n905 = Subtract(x=w1704, y=w1724) -> (x-y=w1723:dbl)
        n906 = Subtract(x=w1726, y=w1724) -> (x-y=w1722:dbl)
        n907 = Subtract(x=w1705, y=w1724) -> (x-y=w1725:dbl)
        n908 = control-ref of="V_DC"() -> (w1706:refnum<vi>)
        n909 = Divide(x=w1725, y=w1722) -> (x/y=w1721:dbl)
        n910 = Divide(x=w1723, y=w1722) -> (x/y=w1719:dbl)
        n911 = Multiply(x=w1721, y=w1717) -> (x*y=w1720:dbl)
        n912 = Multiply(x=w1719, y=w1717) -> (x*y=w1718:dbl)
        n913 = local write "Max Intensity"(w1705) -> ()
        n914 = local write "Min Intensity"(w1704) -> ()
        n915 = property class="IntGraph (strict)"(reference=w1706, error in=w1708, "ZScale.Maximum"=w1705, "ZScale.Minimum"=w1704) -> (error out=w1707:errorcluster)  [unwired: 1 out]
        n916 = local write "Max (%)"(w1720) -> ()
        n917 = local write "Min (%)"(w1718) -> ()
        n918 = local read "Measurement Parameters"() -> (w1740:T4)
        n919 = local read "Bins"() -> (w1730:i32)
        n920 = local read "1w Lifetime (s)"() -> (w1734:dbl[][])
        n921 = local read "DC&1w Lifetime (s)"() -> (w1733:dbl[][])
        n922 = Unbundle By Name(w1740) -> ("Pixel Size"=w1739:dbl)
        n923 = control-ref of="1w Lifetime Hist"() -> (w1732:refnum<vi>)
        n924 = control-ref of="DC&1w Lifetime Hist"() -> (w1731:refnum<vi>)
        n925 = control-ref of="Lifetime Color Ramp"() -> (w1714:refnum<vi>)
        n926 = control-ref of="Composite Image"() -> (w1715:refnum<vi>)
        n927 = To Long Integer(number=w1739) -> (32bit integer=w1713:i32)
        n928 = Square(x=w1713) -> (x^2=w1716:i32)
        n929 = call "LifetimeHistogram.vi"("1w Lifetime"=w1734, "DC&1w Lifetime"=w1733, "1w reference"=w1732, "DC&1w reference"=w1731, "Data Size"=w1716, "error in (no error)"=w1707, "Bins"=w1730) -> ("error out"=w1709:errorcluster, "1w Lifetime Hist"=w1729:T7, "DC&1w Lifetime Hist"=w1728:T7)  [unwired: 6 in, 4 out]
        n930 = call "CompositeProperties.vi"("Image Reference"=w1715, "Ramp Reference"=w1714, "Pixel Size"=w1713, "Max Lifetime (s)"=w1712, "Min Lifetime (s)"=w1711, "error in (no error)"=w1709) -> ("error out"=w1710:errorcluster)  [unwired: 13 in]
        n931 = local write "1w Lifetime Hist"(w1729) -> ()
        n932 = local write "DC&1w Lifetime Hist"(w1728) -> ()
      }
      event "Max (%)", "Min (%)": Value Change {
        w1755 = 100.0 ("y")
        w1780 = 100.0 ("y")
        n933 = event-data() -> ()  [unwired: 1 in, 1 out]
        n934 = local read "V_DC"() -> (w1784:dbl[][])
        n935 = Array Max & Min(array=w1784) -> (max value=w1783:dbl, min value=w1774:dbl)  [unwired: 2 out]
        n936 = Divide(x="Max (%)", y=w1780) -> (x/y=w1779:dbl)
        n937 = Divide(x="Min (%)", y=w1780) -> (x/y=w1778:dbl)
        n938 = Subtract(x=w1783, y=w1774) -> (x-y=w1777:dbl)
        n939 = Multiply(x=w1779, y=w1777) -> (x*y=w1776:dbl)
        n940 = Multiply(x=w1778, y=w1777) -> (x*y=w1775:dbl)
        n941 = Add(x=w1776, y=w1774) -> (x+y=w1766:dbl)
        n942 = Add(x=w1775, y=w1774) -> (x+y=w1765:dbl)
        n943 = local read "Lifetime Selection"() -> (w1773:enum32{"1w Lifetime", "DC&1w Lifetime"})
        n944 = case shown="\"DC&1w Lifetime\"" w1773 {
          tunnel: [w1786 w1787] -> w1770
          frame "1w Lifetime", Default {
            n945 = local read "1w Lifetime (s)"() -> (w1786:dbl[][])
          }
          frame "DC&1w Lifetime" {
            n946 = local read "DC&1w Lifetime (s)"() -> (w1787:dbl[][])
          }
        }
        n947 = local read "Auto Scale?"() -> (w1769:bool)
        n948 = local read "Max Lifetime (s)"() -> (w1768:dbl)
        n949 = local read "V_DC"() -> (w1754:dbl[][])
        n950 = local read "Min Lifetime (s)"() -> (w1767:dbl)
        n951 = call "HSVCombIntensityLifetime.vi"("min_intensity"=w1765, "Auto Scale?"=w1769, "max_intensity"=w1766, "lifetime_max (s)"=w1768, "lifetime_min (s)"=w1767, "Lifetime image"=w1770, "Intensity image"=w1754) -> ("Min"=w1749:dbl, "Max"=w1750:dbl, "Lifetime Color Ramp"=w1772:i32[][], "HSV to RGB Picture"=w1771:picture)  [unwired: 1 in]
        n952 = Array Max & Min(array=w1754) -> (max value=w1764:dbl, min value=w1762:dbl)  [unwired: 2 out]
        n953 = Subtract(x=w1749, y=w1762) -> (x-y=w1761:dbl)
        n954 = Subtract(x=w1764, y=w1762) -> (x-y=w1760:dbl)
        n955 = Subtract(x=w1750, y=w1762) -> (x-y=w1763:dbl)
        n956 = local write "Lifetime Color Ramp"(w1772) -> ()
        n957 = local write "Composite Image"(w1771) -> ()
        n958 = Divide(x=w1763, y=w1760) -> (x/y=w1759:dbl)
        n959 = Divide(x=w1761, y=w1760) -> (x/y=w1757:dbl)
        n960 = control-ref of="V_DC"() -> (w1753:refnum<vi>)
        n961 = Multiply(x=w1759, y=w1755) -> (x*y=w1758:dbl)
        n962 = Multiply(x=w1757, y=w1755) -> (x*y=w1756:dbl)
        n963 = local write "Max (%)"(w1758) -> ()
        n964 = local write "Min (%)"(w1756) -> ()
        n965 = local write "Max Intensity"(w1750) -> ()
        n966 = local write "Min Intensity"(w1749) -> ()
        n967 = property class="IntGraph (strict)"(reference=w1753, error in=w1752, "ZScale.Maximum"=w1750, "ZScale.Minimum"=w1749) -> (error out=w1751:errorcluster)  [unwired: 1 out]
      }
      event "Phasor Plot": Mouse Move; "Phasor Plot": Mouse Down {
        n968 = event-data() -> ("Coords.Horizontal"=w1824:i32, "Coords.Vertical"=w1823:i32, "Type"=w1818:T17)  [unwired: 1 in]
        n969 = control-ref of="Phasor Plot"() -> (w1825:refnum<vi>)
        n970 = property on="Property Node" class="IntGraph (strict)"(reference=w1825, error in=w1844, "Width"="PicSize", "Height"="PicSize") -> (error out=w1813:errorcluster, "XScale.Maximum"=w1843:dbl, "XScale.Minimum"=w1837:dbl, "YScale.Maximum"=w1832:dbl, "YScale.Minimum"=w1833:dbl, "Plot Bounds"=w1836:T18)  [unwired: 1 out]
        n971 = Unbundle By Name(w1836) -> ("Left"=w1842:i16, "Top"=w1835:i16)
        n972 = Subtract(x=w1824, y=w1842) -> (x-y=w1820:i32)
        n973 = Subtract(x=w1823, y=w1835) -> (x-y=w1819:i32)
        n974 = Subtract(x=w1843, y=w1837) -> (x-y=w1841:dbl)
        n975 = Subtract(x=w1832, y=w1833) -> (x-y=w1840:dbl)
        n976 = Divide(x=w1841, y="PicSize") -> (x/y=w1839:dbl)
        n977 = Divide(x=w1840, y="PicSize") -> (x/y=w1834:dbl)
        n978 = Multiply(x=w1820, y=w1839) -> (x*y=w1838:dbl)
        n979 = Multiply(x=w1819, y=w1834) -> (x*y=w1831:dbl)
        n980 = Add(x=w1838, y=w1837) -> (x+y=w1809:dbl)
        "G" <- w1809
        n981 = Subtract(x=w1832, y=w1831) -> (x-y=w1808:dbl)
        "S" <- w1808
        n982 = Bundle(w1809, w1808) -> (w1821:cluster{dbl, dbl})  [unwired: 1 in]
        n983 = Multiply(x=80000000.0, y=6.283185307179586) -> (x*y=w1827:dbl)
        n984 = Divide(x=w1808, y=w1809) -> (x/y=w1828:dbl)
        n985 = Divide(x=w1828, y=w1827) -> (x/y=→"[tau]":dbl)
        n986 = case shown="\"ROI1\", Default" "ROI Select" {
          tunnel: [w1845 w1846 w1847 w1848] -> w1815
          frame "ROI1", Default {
            n987 = local read "Center1"() -> (w1845:cluster{dbl, dbl})
          }
          frame "ROI2" {
            n988 = local read "Center2"() -> (w1846:cluster{dbl, dbl})
          }
          frame "ROI3" {
            n989 = local read "Center3"() -> (w1847:cluster{dbl, dbl})
          }
          frame "ROI4" {
            n990 = local read "Center4"() -> (w1848:cluster{dbl, dbl})
          }
        }
        n991 = property on="Phasor Plot" class="IntGraph (strict)"(error in=w1813) -> (error out=w1812:errorcluster, "PlotImages.Front"=w1811:picture)  [unwired: 1 in, 1 out]
        n992 = local read "Radius4"() -> (w1796:dbl)
        n993 = local read "Center4"() -> (w1795:cluster{dbl, dbl})
        n994 = local read "Radius2"() -> (w1800:dbl)
        n995 = local read "Center2"() -> (w1799:cluster{dbl, dbl})
        n996 = local read "Radius3"() -> (w1798:dbl)
        n997 = local read "Center3"() -> (w1797:cluster{dbl, dbl})
        n998 = local read "Radius1"() -> (w1802:dbl)
        n999 = local read "Center1"() -> (w1801:cluster{dbl, dbl})
        n1000 = local read "PicSize"() -> (w1794:u32)
        n1001 = case shown="\"Mouse Move\", Default" w1818 {
          tunnel: w1821 -> [w1851 w1888]
          tunnel: [w1853 w1889] -> w1817
          tunnel: w1812 -> [w1854 w1890]
          tunnel: [w1854 w1890] -> w1816
          tunnel: w1815 -> [_ w1887]
          tunnel: w1811 -> [w1853 w1885]
          tunnel: "ROI Select" -> [w1852 w1884]
          tunnel: w1802 -> [_ w1883]
          tunnel: w1801 -> [_ w1882]
          tunnel: "Color1" -> [_ w1881]
          tunnel: w1800 -> [_ w1880]
          tunnel: w1799 -> [_ w1879]
          tunnel: "Color2" -> [_ w1878]
          tunnel: w1798 -> [_ w1877]
          tunnel: w1797 -> [_ w1876]
          tunnel: "Color3" -> [_ w1875]
          tunnel: w1796 -> [_ w1874]
          tunnel: w1795 -> [_ w1873]
          tunnel: "Color4" -> [_ w1872]
          tunnel: "ROI4?" -> [_ w1871]
          tunnel: "ROI2?" -> [_ w1870]
          tunnel: "ROI1?" -> [_ w1869]
          tunnel: w1794 -> [_ w1868]
          tunnel: "ROI3?" -> [_ w1867]
          frame "Mouse Down" {
            w1849 = TRUE ("ROI Drawing")
            n1002 = case shown="\"ROI4\"" w1852 {
              tunnel: w1851 -> [_ w1857 w1860 w1863 w1866]
              tunnel: 0.0 ("Radius2") -> [_ w1856 w1859 w1862 w1865]
              tunnel: w1849 -> [_ w1855 w1858 w1861 w1864]
              frame "None" {
              }
              frame "ROI1" {
                n1003 = local write "Radius1"(w1856) -> ()
                n1004 = local write "ROI1?"(w1855) -> ()
                "Center1" <- w1857
              }
              frame "ROI2" {
                n1005 = local write "Radius2"(w1859) -> ()
                n1006 = local write "ROI2?"(w1858) -> ()
                "Center2" <- w1860
              }
              frame "ROI3" {
                n1007 = local write "Radius3"(w1862) -> ()
                n1008 = local write "ROI3?"(w1861) -> ()
                "Center3" <- w1863
              }
              frame "ROI4" {
                n1009 = local write "Radius4"(w1865) -> ()
                n1010 = local write "ROI4?"(w1864) -> ()
                "Center4" <- w1866
              }
            }
            "ROI Drawing" <- w1849
          }
          frame "Mouse Move", Default {
            n1011 = local read "ROI Drawing"() -> (w1886:bool)
            n1012 = case shown="True" w1886 {
              tunnel: [w1891 w1913] -> w1889
              tunnel: w1888 -> [_ w1927]
              tunnel: w1887 -> [_ w1926]
              tunnel: w1885 -> [w1891 _]
              tunnel: w1884 -> [_ w1918]
              tunnel: w1883 -> [_ w1911]
              tunnel: w1882 -> [_ w1910]
              tunnel: w1881 -> [_ w1909]
              tunnel: w1880 -> [_ w1908]
              tunnel: w1879 -> [_ w1898]
              tunnel: w1878 -> [_ w1906]
              tunnel: w1877 -> [_ w1905]
              tunnel: w1876 -> [_ w1897]
              tunnel: w1875 -> [_ w1904]
              tunnel: w1874 -> [_ w1901]
              tunnel: w1873 -> [_ w1900]
              tunnel: w1872 -> [_ w1899]
              tunnel: w1871 -> [_ w1902]
              tunnel: w1870 -> [_ w1907]
              tunnel: w1869 -> [_ w1912]
              tunnel: w1868 -> [_ w1916]
              tunnel: w1867 -> [_ w1892]
              frame False {
              }
              frame True {
                n1013 = Subtract(x=w1926, y=w1927) -> (x-y=w1925:cluster{dbl, dbl})
                n1014 = call "Empty Picture"() -> ("empty picture"=w1917:picture)
                n1015 = Unbundle(w1925) -> (w1924:dbl, w1923:dbl)